vi "UHR-Fleezers Control (host) - 12.8.vi"() -> ()   [LabVIEW 2012] (continued)
        n3045 = xnode "Read/Write Control"("FPGA VI Reference In"=w4146, "error in"=w4145) -> ("FPGA VI Reference Out"=w4144:T20, "error out"=w4143:errorcluster, "APD 3 Gate Late Counter"=→"APD 3 Gate Late Counter":u8, "APD 3 Gate Relative Phase"=→"APD 3 Gate Relative Phase":i16)
      }
    }
    n3046 = Not Equal?(x=w3817, y="Calibration") -> (x != y?=w3778:bool)
    n3047 = case shown="True" w3778 {
      tunnel: w3815 -> [_ w4177]
      tunnel: w3814 -> [_ w4176]
      tunnel: w3813 -> [_ w4175]
      tunnel: w3810 -> [_ w4174]
      tunnel: w3754 -> [_ w4173]
      frame False {
      }
      frame True {
        n3048 = property on="Force" class="WFChart (strict)"("YScale.NameLbl.Text"=w4177) -> ()  [unwired: 2 in, 2 out]
        n3049 = property on="T2 X" class="DigNum (strict)"("Caption.Text"=w4175) -> ()  [unwired: 2 in, 2 out]
        n3050 = property on="T1 X" class="DigNum (strict)"("Caption.Text"=w4176) -> ()  [unwired: 2 in, 2 out]
        n3051 = property on="Mean" class="DigNum (strict)"("Caption.Text"=w4174) -> ()  [unwired: 2 in, 2 out]
        n3052 = property on="Difference" class="DigNum (strict)"("Caption.Text"=w4173) -> ()  [unwired: 2 in, 2 out]
      }
    }
    n3053 = Unbundle By Name(w3553) -> ("Y"=w3801:dbl[])
    n3054 = Unbundle By Name(w3552) -> ("Y"=w3804:dbl[])
    n3055 = Subtract(x=w3801, y=w3799) -> (x-y=w3802:dbl[])
    n3056 = Subtract(x=w3804, y=w3798) -> (x-y=w3803:dbl[])
    n3057 = Multiply(x=w3803, y="T2 alpha_x (nm/V)") -> (x*y=w3603:dbl[])
    n3058 = Multiply(x="T1 alpha_x (nm/V)", y=w3802) -> (x*y=w3604:dbl[])
    n3059 = Not(x="Trap Trig. Fl.") -> (.not. x?=w3640:bool)
    n3060 = Multiply(x=w3825, y=-1.0) -> (x*y=w3806:waveform(dbl))
    n3061 = Subtract(x=w3604, y=w3603) -> (x-y=w3796:dbl[])
    n3062 = Unbundle By Name(w3825) -> ("Y"=w3769:dbl[])
    n3063 = Unbundle By Name(w3826) -> ("Y"=w3605:dbl[])
    n3064 = Negate(x=w3796) -> (-x=w3601:dbl[])
    n3065 = Build Array(w3826, w3806) -> (→"Force":waveform(dbl)[])
    n3066 = Subtract(x=w3601, y="Offset (nm)") -> (x-y=w3768:dbl[])
    n3067 = call-poly <vilib>:"Mean.vi"("X"=w3769) -> ("mean"=w3607:dbl)  [unwired: 1 out]
    "T2 X" <- w3607
    n3068 = Negate(x=w3769) -> (-x=w3546:dbl[])
    n3069 = call-poly <vilib>:"Mean.vi"("X"=w3605) -> ("mean"=w3608:dbl)  [unwired: 1 out]
    "T1 X" <- w3608
    n3070 = Negate(x=w3607) -> (-x=w3606:dbl)
    n3071 = Bundle By Name(cluster=w3553, "Y"=w3768) -> (w3746:waveform(dbl))
    "Bead Separation" <- w3746
    n3072 = Add(x=w3605, y=w3546) -> (x+y=w3770:dbl[])
    n3073 = Divide(x=w3770, y=2.0) -> (x/y=w3549:dbl[])
    n3074 = Add(x=w3608, y=w3606) -> (x+y=w3812:dbl)
    n3075 = Subtract(x=w3608, y=w3606) -> (x-y=→"Difference":dbl)
    n3076 = Select(t=w3546, s="Only check fixed trap T2", f=w3549) -> (s? t:f=→"Vec Mean of T1 T2":dbl[])
    n3077 = Divide(x=w3812, y=2.0) -> (x/y=w3772:dbl)
    "Mean" <- w3772
    n3078 = feedback-in #25("Trap Trig. Fl.") -> ()
    n3079 = feedback #25("Trap Trig. Fl.") -> (w3638:bool)
    n3080 = And(x=w3640, y=w3638) -> (x .and. y?=w3639:bool)
    n3081 = case "If have just turned off triggering" shown="True" w3639 {
      tunnel: w3621 -> [_ w3974]
      tunnel: w3620 -> [_ w3973]
      frame False {
      }
      frame True {
        w3972 = FALSE ("FPGA Trap Trig")
        n3082 = xnode "Read/Write Control"("FPGA VI Reference In"=w3974, "error in"=w3973, "FPGA Trap Trig"=w3972) -> ("FPGA VI Reference Out"=w3971:T20, "error out"=w3970:errorcluster)
        n3083 = xnode "Read/Write Control"("FPGA VI Reference In"=w3971, "error in"=w3970, "TTrig?"=w3972) -> ()  [unwired: 2 out]
        n3084 = local write "Initializing"(FALSE ("Initializing")) -> ()
        n3085 = local write "Triggered"(FALSE ("Triggered")) -> ()
        n3086 = local write "Waiting"(FALSE ("Waiting")) -> ()
      }
    }
    n3087 = Not(x=w3638) -> (.not. x?=w3651:bool)
    n3088 = And(x="Trap Trig. Fl.", y=w3651) -> (x .and. y?=w3648:bool)
    n3089 = local read "Tether"() -> (w3773:bool)
    n3090 = Or(x=w3648, y="Reinitialize") -> (x .or. y?=w3634:bool)
    n3091 = feedback #26(w3644) -> (w3649:string)
    n3092 = Select(t=w3644, s=w3648, f=w3649) -> (s? t:f=w3643:string)
    n3093 = Select(t=w3644, s="Reinitialize", f=w3643) -> (s? t:f=w3642:string)
    n3094 = feedback #27(0) -> (w3646:i32)
    n3095 = feedback #28(w3768) -> (w3767:dbl[])
    n3096 = Build Array (concatenate)(w3768, w3767) -> (w3602:dbl[])
    n3097 = case "For determining if there is a tether still" shown="True" w3773 {
      tunnel: w3772 -> [_ w4098]
      frame False {
      }
      frame True {
        n3098 = Greater?(x="Lost Tether Alarm Threshold (pN)", y=w4098) -> (0:w4096:bool)
        n3099 = case shown="True" w4096 {
          frame False {
          }
          frame True {
            w4099 = FALSE ("Value (Signaling)")
            n3100 = flat-sequence {
              frame #0 {
                # "stop only if saving"
                n3101 = local read "Saving..."() -> (w4111:bool)
                n3102 = And(x=w4111, y="TA Cancel Save?") -> (x .and. y?=w4110:bool)
                n3103 = local write "Stop Saving"(w4110) -> ()
              }
              frame #1 {
                n3104 = case shown="True" "TA Green Off?" {
                  frame False {
                  }
                  frame True {
                    w4114 = FALSE ("Fl. Triggered...")
                    n3105 = local write "Fl. Triggered..."(w4114) -> ()
                    n3106 = property on="Green Laser ON" class="Bool (strict)"("Val(Sgnl)"=w4114) -> ()  [unwired: 2 in, 2 out]
                  }
                }
              }
            }
            n3107 = local read "Time tether formed"() -> (w4105:timestamp)
            n3108 = Get Date/Time In Seconds() -> (seconds since 1Jan1904=w4106:timestamp)
            n3109 = Subtract(x=w4106, y=w4105) -> (x-y=w4104:dbl)
            n3110 = Number To Decimal String(number=w4104) -> (decimal integer string=w4101:string)  [unwired: 1 out]
            n3111 = local read "Messages"() -> (w4108:string)
            n3112 = call <vilib>:"Beep.vi"() -> ()  [unwired: 3 in, 9 out]
            n3113 = Concatenate Strings("Lost tether (" ("Message to add"), w4101, " s)." ("string")) -> (w4103:string)
            n3114 = local write "Tether"(FALSE ("Tether")) -> ()
            n3115 = call "Update messages.vi"("Message to add"=w4103, "Old message string"=w4108) -> ("New message string"=w4107:string)
            n3116 = local write "Messages"(w4107) -> ()
            n3117 = property on="Fl. Triggered..." class="Bool (strict)"("Val(Sgnl)"=w4099) -> ()  [unwired: 2 in, 2 out]
            n3118 = local write "Dip for Protein"(w4099) -> ()
            n3119 = property on="Trap Pos. FB ON" class="Bool (strict)"("Val(Sgnl)"=w4099) -> ()  [unwired: 2 in, 2 out]
            n3120 = property on="Trap Trig. Fl." class="Bool (strict)"("Val(Sgnl)"=w4099) -> ()  [unwired: 2 in, 2 out]
          }
        }
      }
    }
    n3121 = case "For triggering actions based on the trap position (e.g., turning the excitation laser on if trap under feedback moves so far)" shown="True" "Trap Trig. Fl." {
      tunnel: w3629 -> [_ w3987]
      tunnel: w3642 -> [_ w3986]
      tunnel: ["" ("t") w3985] -> w3650
      tunnel: w3634 -> [_ w3984]
      tunnel: [0 ("t") w3983] -> w3647
      tunnel: w3646 -> [_ w3982]
      tunnel: w3621 -> [_ w3981]
      tunnel: w3620 -> [_ w3980]
      frame False {
      }
      frame True {
        n3122 = case shown="\"Wait for trigger\"" w3986 {
          tunnel: w3987 -> [w4004 _ _ w4052]
          tunnel: [w4001 w4033 "" ("t") w4055] -> w3985
          tunnel: w3984 -> [_ _ _ w4043]
          tunnel: [w4000 w4030 0 ("t") w4044] -> w3983
          tunnel: w3982 -> [_ w4032 _ w4050]
          tunnel: w3981 -> [w3989 w4027 _ w4046]
          tunnel: w3980 -> [w3988 w4026 _ w4045]
          frame "Wait for trigger" {
            n3123 = local read "Trap Trig. (FPGA)"() -> (w3992:bool)
            n3124 = Subtract(x=w4004, y="Mean T1 Position\nto compare (nm)") -> (x-y=w3997:dbl[])
            n3125 = call <vilib>:"Std Deviation and Variance.vi"("X"=w3997) -> ("mean"=→"mean":dbl, "standard deviation"=→"standard\ndeviation":dbl)  [unwired: 1 in, 1 out]
            n3126 = Array Max & Min(array=w3997) -> (max value=→"max value":dbl, min value=→"min value":dbl)  [unwired: 2 out]
            n3127 = Greater?(x=w3997, y="Threshold (nm)") -> (0:w4007:bool[])
            n3128 = case shown="True" w3992 {
              tunnel: w3989 -> [_ w4013]
              tunnel: w3988 -> [_ w4012]
              tunnel: [FALSE ("TTrig?") w4011] -> w3995
              frame False {
              }
              frame True {
                n3129 = xnode "Read/Write Control"("FPGA VI Reference In"=w4013, "error in"=w4012) -> ("TTrig?"=w4011:bool)  [unwired: 2 out]
              }
            }
            n3130 = Or Array Elements(Boolean array=w4007) -> (logical OR=w3994:bool)
            n3131 = Select(t=w3995, s=w3992, f=w3994) -> (s? t:f=w3993:bool)
            n3132 = Not(x=w3992) -> (.not. x?=w3991:bool)
            n3133 = And(x=w3993, y=w3991) -> (x .and. y?=w3990:bool)
            n3134 = Select(t="Triggered", s=w3993, f="Wait for trigger") -> (s? t:f=w4001:string)
            n3135 = case shown="True" w3993 {
              tunnel: [0 0] -> w4000
              tunnel: w3989 -> [_ w4018]
              tunnel: w3988 -> [_ w4017]
              frame False {
                "Waiting" <- TRUE ("Waiting")
              }
              frame True {
                n3136 = xnode "Read/Write Control"("FPGA VI Reference In"=w4018, "error in"=w4017, "TTrig?"=FALSE) -> ()  [unwired: 2 out]
                n3137 = local read "Messages"() -> (w4021:string)
                n3138 = call <vilib>:"Beep.vi"() -> ()  [unwired: 12 in]
                n3139 = call "Update messages.vi"("Message to add"="Unwinding trigger.", "Old message string"=w4021) -> ("New message string"=w4022:string)
                n3140 = local write "Messages"(w4022) -> ()
                n3141 = local write "Waiting"(FALSE ("Waiting")) -> ()
                "Triggered" <- TRUE ("Triggered")
              }
            }
            n3142 = case "Only need to turn on laser if host triggered" shown="True" w3990 {
              frame False {
              }
              frame True {
                n3143 = property on="Green Laser ON" class="Bool (strict)"("Val(Sgnl)"=TRUE ("Value (Signaling)")) -> ()  [unwired: 2 in, 2 out]
              }
            }
          }
          frame "Triggered" {
            n3144 = local read "Trap Trig. (FPGA)"() -> (w4029:bool)
            n3145 = Increment(x=w4032) -> (x+1=w4030:i32)
            n3146 = Greater Or Equal?(x=w4030, y="Fl. ON time (n)") -> (x >= y?=w4028:bool)
            n3147 = Select(t="Wait for trigger", s=w4028, f="Triggered" ("t")) -> (s? t:f=w4033:string)
            n3148 = And(x=w4028, y=w4029) -> (x .and. y?=w4025:bool)
            n3149 = case shown="True" w4025 {
              tunnel: w4027 -> [_ w4037]
              tunnel: w4026 -> [_ w4036]
              frame False {
              }
              frame True {
                n3150 = xnode "Read/Write Control"("FPGA VI Reference In"=w4037, "error in"=w4036, "FPGA Trap Trig"=TRUE) -> ()  [unwired: 2 out]
              }
            }
            n3151 = case shown="True" w4028 {
              frame False {
              }
              frame True {
                w4039 = FALSE ("Value (Signaling)")
                n3152 = local write "Triggered"(w4039) -> ()
                n3153 = local write "Waiting"(TRUE ("Waiting")) -> ()
                n3154 = property on="Green Laser ON" class="Bool (strict)"("Val(Sgnl)"=w4039) -> ()  [unwired: 2 in, 2 out]
              }
            }
          }
          frame "Do nothing" {
          }
          frame "Initialize", Default {
            n3155 = Increment(x=w4050) -> (x+1=w4054:i32)
            n3156 = Select(t=1, s=w4043, f=w4054) -> (s? t:f=w4044:i32)
            n3157 = feedback #29(w4052) -> (w4058:dbl[])
            n3158 = Build Array (concatenate)(w4052, w4058) -> (w4051:dbl[])
            n3159 = Greater Or Equal?(x=w4044, y="Wait to get offset (n)") -> (x >= y?=w4047:bool)
            n3160 = Select(t=w4052, s=w4043, f=w4051) -> (s? t:f=w4053:dbl[])
            n3161 = feedback-in #29(w4053) -> ()
            n3162 = call-poly <vilib>:"Mean.vi"("X"=w4053) -> ("mean"=w4048:dbl)  [unwired: 1 out]
            n3163 = local write "Mean T1 Position\nto compare (nm)"(w4048) -> ()
            n3164 = case shown="True" w4043 {
              tunnel: w4046 -> [_ w4064]
              tunnel: w4045 -> [_ w4063]
              frame False {
              }
              frame True {
                w4060 = FALSE ("FPGA Trap Trig")
                n3165 = xnode "Read/Write Control"("FPGA VI Reference In"=w4064, "error in"=w4063, "FPGA Trap Trig"=w4060) -> ("FPGA VI Reference Out"=w4062:T20, "error out"=w4061:errorcluster)
                n3166 = xnode "Read/Write Control"("FPGA VI Reference In"=w4062, "error in"=w4061, "TTrig?"=w4060) -> ()  [unwired: 2 out]
              }
            }
            n3167 = Select(t="Wait for trigger", s=w4047, f="Initialize") -> (s? t:f=w4055:string)
            n3168 = case shown="True" w4047 {
              tunnel: w4048 -> [_ w4067]
              tunnel: w4046 -> [_ w4076]
              tunnel: w4045 -> [_ w4075]
              frame False {
                n3169 = local write "Waiting"(FALSE ("Waiting")) -> ()
                "Initializing" <- TRUE ("Initializing")
              }
              frame True {
                n3170 = local read "Threshold (nm)"() -> (w4079:dbl)
                n3171 = local read "AOM X Cal (nm/MHz)"() -> (w4078:dbl)
                n3172 = Add(x=w4067, y=w4079) -> (x+y=w4080:dbl)
                n3173 = Divide(x=w4080, y=w4078) -> (x/y=w4077:dbl)
                n3174 = call "IR AOM freq to word.vi"("Frequency In (MHz)"=w4077) -> ("Frequency Word Out (double)"=w4074:dbl)
                n3175 = local write "Initializing"(FALSE ("Initializing")) -> ()
                n3176 = local write "Waiting"(TRUE ("Waiting")) -> ()
                n3177 = To Quad Integer(1:w4074) -> (0:w4073:i64)
                n3178 = xnode "Read/Write Control"("FPGA VI Reference In"=w4076, "error in"=w4075, "FPGA TTrig Thresh"=w4073) -> ("FPGA VI Reference Out"=w4070:T20, "error out"=w4069:errorcluster)
                n3179 = xnode "Read/Write Control"("FPGA VI Reference In"=w4070, "error in"=w4069, "FPGA Trap Trig"=TRUE) -> ()  [unwired: 2 out]
              }
            }
          }
        }
      }
    }
    n3180 = feedback-in #26(w3650) -> ()
    n3181 = feedback-in #27(w3647) -> ()
    n3182 = Split 1D Array(array=w3602, index=w3664) -> (first subarray=w3764:dbl[])  [unwired: 1 out]
    n3183 = feedback-in #28(w3764) -> ()
    n3184 = call-poly <vilib>:"Mean.vi"("X"=w3764) -> ("mean"=w3763:dbl)  [unwired: 1 out]
    "Bead Mean (nm)" <- w3763
    n3185 = Subtract(x=w3764, y=w3763) -> (x-y=w3762:dbl[])
    n3186 = Square(x=w3762) -> (x^2=w3761:dbl[])
    n3187 = call-poly <vilib>:"Mean.vi"("X"=w3761) -> ("mean"=w3760:dbl)  [unwired: 1 out]
    n3188 = Square Root(x=w3760) -> (sqrt(x)=w3759:dbl)
    n3189 = Multiply(x=10.0, y=w3759) -> (x*y=→"RMS (Ang)":dbl)
    n3190 = xnode ("Read/Write Control")("FPGA VI Reference In"=w3794, "error in"=w3793) -> ("FPGA VI Reference Out"=w3632:T20, "error out"=w3631:errorcluster, "AI2 Y Sum Set 1"=w3887:i16, "AI2 Y Sum Set 2"=w3886:i16, "AI1 X Set 1"=w3696:fxp<+/-,16,1>, "AI1 X Set 2"=w3695:fxp<+/-,16,1>, "Trap Pos FB Int Signal"=→"Trap Pos FB Int Signal":fxp<+/-,24,9>, "Trap Pos FB Int-Norm Signal"=→"Trap Pos FB Int-Norm Signal":fxp<+/-,16,1>, "Trap Pos FB Action"=w3689:i64, "Scanning"=→"AOD Scanning":bool, "Scan I"=→"AOD Scan I":u64, "Scanning MCL"=w3889:bool, "Scan I (MCL)"=→"MCL Scan I":u64, "Green FB Sum"=w3829:i16, "Trap Pos FB Action"=w3619:i64, "TTrig Fin Thresh"=w3615:i64, "Red FB Intensity"=w3596:i16, "Blue Intensity"=w3591:i16)
    "MCL Scanning" <- w3889
    "Trap Pos FB Action" <- w3689
    n3191 = Divide(x=w3596, y=3276.7) -> (x/y=w3595:dbl)
    "Red laser intensity (V)" <- w3595
    n3192 = Divide(x=w3591, y=3276.7) -> (x/y=w3590:dbl)
    "Blue laser intensity (V)" <- w3590
    n3193 = Divide(x=w3829, y=3276.7) -> (x/y=w3594:dbl)
    "Green laser intensity (V)" <- w3594
    n3194 = local read "FB Trig Integrate"() -> (w3613:u32)
    n3195 = Divide(x=w3619, y=w3613) -> (x/y=w3612:dbl)
    "TTrig Sig (Int)" <- w3612
    n3196 = Bundle(w3594, w3595, w3590) -> (→"Fluorescence laser intensities plot":cluster{dbl, dbl, dbl})  [unwired: 1 in]
    n3197 = Divide(x=w3615, y=w3613) -> (x/y=w3610:dbl)
    "TTrig Fin Thresh (Int)" <- w3610
    n3198 = local read "AOM X Cal (nm/MHz)"() -> (w3618:dbl)
    n3199 = local read "AI2 (V)"() -> (w3888:cluster{"Set 1":dbl, "Set 2":dbl})
    n3200 = Bundle By Name(cluster=w3888, "Set 1"=w3887, "Set 2"=w3886) -> (w3884:cluster{"Set 1":dbl, "Set 2":dbl})
    n3201 = Divide(x=w3689, y=327.67) -> (x/y=→"Action (%)":dbl)
    n3202 = local read "Trap X (AI1)"() -> (w3709:T10)
    n3203 = call "IR AOM word double to freq.vi"("Frequency Word In (double)"=w3610) -> ("Frequency Out (MHz)"=w3609:dbl)
    n3204 = call "IR AOM word double to freq.vi"("Frequency Word In (double)"=w3612) -> ("Frequency Out (MHz)"=w3611:dbl)
    n3205 = Divide(x=w3884, y=3276.7) -> (x/y=w3883:cluster{"Set 1":dbl, "Set 2":dbl})
    n3206 = Multiply(x=w3611, y=w3618) -> (x*y=w3617:dbl)
    "TTrig Sig (nm)" <- w3617
    n3207 = Multiply(x=w3609, y=w3618) -> (x*y=w3616:dbl)
    "TTrig Fin Thresh (nm)" <- w3616
    n3208 = local write "AI2 (V)"(w3883) -> ()
    n3209 = Bundle(cluster=w3709, "Trap 1"=w3696, "Trap 2"=w3695) -> (→"Trap X (AI1)":T10)
    n3210 = Bundle(w3617, w3616) -> (→"TTrig":cluster{dbl, dbl})  [unwired: 1 in]
    n3211 = flat-sequence "To save data" {
      tunnel: [w4998] -> w3907
      tunnel: [w4999] -> w3906
      tunnel: w3858 -> [w4992]
      tunnel: w3637 -> [w4996]
      tunnel: ["Save Calibration"] -> w3880
      tunnel: w3877 -> [w4995]
      tunnel: [w4988] -> w3876
      tunnel: [w4985] -> w3875
      tunnel: [w4982] -> w3874
      tunnel: w3857 -> [w4984]
      tunnel: w3776 -> [w4978]
      tunnel: [w4978] -> w3775
      tunnel: [w4970] -> w3747
      tunnel: [w4973] -> w3677
      tunnel: [w4972] -> w3676
      tunnel: w3907 -> [w5248]
      tunnel: w3906 -> [w5247]
      tunnel: w3678 -> [w5246]
      tunnel: w3880 -> [w5245]
      tunnel: w3876 -> [w5243]
      tunnel: w3875 -> [w5242]
      tunnel: w3874 -> [w5241]
      tunnel: w3756 -> [w5240]
      tunnel: w3786 -> [w5239]
      tunnel: w3775 -> [w5238]
      tunnel: w3747 -> [w5237]
      tunnel: w3746 -> [w5236]
      tunnel: w3576 -> [w5235]
      tunnel: w3677 -> [w5234]
      tunnel: w3676 -> [w5233]
      tunnel: w3675 -> [w5232]
      tunnel: w3598 -> [w5231]
      frame #0 {
        n3212 = Or(x="Start Saving", y="Start saving data + video") -> (x .or. y?=w4970:bool)
        n3213 = case shown="True" "Start saving data + video" {
          frame False {
          }
          frame True {
            n3214 = stacked-sequence {
              frame #0 {
                n3215 = local write "New Video File"(TRUE ("New Video File")) -> ()
              }
              frame #1 {
                n3216 = local write "Save Video"(TRUE ("Save Video")) -> ()
              }
            }
          }
        }
        n3217 = Or(x="Save N Sets", y=w4970) -> (x .or. y?=w4979:bool)
        n3218 = To Double Precision Float(number=w4995) -> (double precision float=w4989:dbl)
        n3219 = Build Array(w4979, "Save Calibration", w4992, w4984) -> (w4994:bool[])
        n3220 = Compound Arithmetic op=OR("Save Calibration", w4992, w4979, w4984) -> (w4997:bool)
        n3221 = Boolean Array To Number(Boolean array=w4994) -> (number=w4991:u32)
        n3222 = feedback #30(FALSE ("Save APD Data\nwith Trap Data")) -> (w4974:bool)
        n3223 = feedback #31(refnum<k0> refnum) -> (w5000:refnum<file>)
        n3224 = feedback #32(refnum<k0> refnum) -> (w4976:refnum<file>)
        n3225 = feedback #33(FALSE ("Save APD Data\nwith Trap Data")) -> (w4983:bool)
        n3226 = feedback #34(refnum<k0> refnum) -> (w4986:refnum<file>)
        n3227 = feedback #35(0) -> (w5002:i32)
        n3228 = feedback #36() -> (w4990:u32)  [unwired: 1 out]
        n3229 = case shown="True" w4997 {
          tunnel: [w5011 1] -> w4998
          tunnel: w5002 -> [w5013 _]
          tunnel: [w5012 w5044] -> w4999
          tunnel: w5000 -> [w5012 _]
          tunnel: w4996 -> [_ w5062]
          tunnel: w4989 -> [_ w5060]
          tunnel: w4991 -> [_ w5063]
          tunnel: [w5010 w5043] -> w4988
          tunnel: w4990 -> [w5010 _]
          tunnel: [w5009 w5041] -> w4985
          tunnel: w4986 -> [w5009 _]
          tunnel: [w5008 w5040] -> w4982
          tunnel: w4983 -> [w5008 _]
          tunnel: w4970 -> [_ w5038]
          tunnel: w4978 -> [_ w5037]
          tunnel: [w5007 w5029] -> w4972
          tunnel: w4976 -> [w5007 _]
          tunnel: [w5006 w5028] -> w4973
          tunnel: w4974 -> [w5006 _]
          frame False {
            n3230 = Increment(x=w5013) -> (x+1=w5011:i32)
          }
          frame True {
            w5034 = FALSE ("Start Saving")
            w5039 = 9.0  # File Version
            w5046 = FALSE ("prepend array or string size? (T)")
            w5045 = T28."big-endian, network order" ("byte order (0:big-endian, network order)")
            n3231 = local read "BD 1 Frequency 1 (MHz)"() -> (w5059:dbl)
            n3232 = local read "BD 2 Frequency 1 (MHz)"() -> (w5058:dbl)
            n3233 = local read "BD 1 Frequency 2 (MHz)"() -> (w5057:dbl)
            n3234 = local read "BD 2 Frequency 2 (MHz)"() -> (w5056:dbl)
            n3235 = local read "BD 1 Frequency 3 (MHz)"() -> (w5055:dbl)
            n3236 = local read "BD 2 Frequency 3 (MHz)"() -> (w5054:dbl)
            n3237 = Array Size(array=w5037) -> (size(s)=w5036:i32)
            n3238 = To Double Precision Float(number=w5036) -> (double precision float=w5035:dbl)
            n3239 = local write "Save Calibration"(w5034) -> ()
            n3240 = local write "Start Saving"(w5034) -> ()
            n3241 = Build Array("Save APD Data\nwith Trap Data", "Save Trap Pos. Data") -> (w5031:bool[])
            n3242 = Boolean Array To Number(Boolean array=w5031) -> (number=w5030:u32)
            n3243 = Build Array(w5059, w5058, w5057, w5056, w5055, w5054) -> (w5053:dbl[])
            n3244 = case shown="1, Default" w5063 {
              tunnel: w5062 -> [w5135 w5155 w5171 w5209]
              tunnel: w5035 -> [w5140 w5162 w5191 w5228]
              tunnel: w5060 -> [w5139 w5161 w5190 w5227]
              tunnel: [w5136 w5157 w5182 w5219] -> w5051
              tunnel: [w5127 "Cal sets to save" w5172 w5210] -> w5043
              tunnel: w5053 -> [w5137 w5158 w5184 w5221]
              tunnel: "Save APD Data\nwith Trap Data" -> [w5134 _ w5168 w5207]
              tunnel: [w5134 w5149 w5168 w5207] -> w5040
              tunnel: w5039 -> [w5130 w5150 w5166 w5205]
              tunnel: w5038 -> [w5129 _ _ _]
              tunnel: [w5120 w5149 w5165 w5195] -> w5028
              tunnel: "Save Trap Pos. Data" -> [w5120 _ w5165 w5195]
              tunnel: w5030 -> [w5119 _ w5164 w5194]
              frame 1, Default {
                # "timeseries"
                n3245 = case shown="True" "Profile" {
                  tunnel: [w5143 w5147] -> w5124
                  tunnel: [w5143 w5146] -> w5123
                  tunnel: [w5143 w5145] -> w5122
                  tunnel: [w5143 w5144] -> w5121
                  frame False {
                    w5143 = 0.0 ("f")
                  }
                  frame True {
                    n3246 = local read "Current Position"() -> (w5148:cluster{dbl, dbl, dbl})
                    n3247 = local read "Y change (mm)"() -> (w5144:dbl)
                    n3248 = Unbundle(w5148) -> (w5147:dbl, w5146:dbl, w5145:dbl)
                  }
                }
                n3249 = local read "Save ave N"() -> (w5142:dbl)
                n3250 = Multiply(x=w5142, y=w5135) -> (x*y=w5141:dbl)
                n3251 = To Double Precision Float(number=w5119) -> (double precision float=w5133:dbl)
                n3252 = Build Array(w5130, w5135, w5141, w5140, w5139, 0.0 ("f")) -> (w5138:dbl[])
                n3253 = Build Array(w5133, w5124, w5123, w5122, w5121) -> (w5131:dbl[])
                n3254 = Select(t=u32 4000000000, s=w5129, f="N sets to save") -> (s? t:f=w5127:u32)
                n3255 = Build Array (concatenate)(w5138, w5137, w5131) -> (w5136:dbl[])
              }
              frame 2 {
                w5152 = 0.0 ("f")
                w5149 = FALSE ("Save APD Data\nwith Trap Data")
                # "calibration"
                n3256 = Boolean To (0,1)(Boolean=w5149) -> (0, 1=w5154:i16)
                n3257 = To Double Precision Float(number=w5154) -> (double precision float=w5153:dbl)
                n3258 = Build Array(w5153, w5152, w5152, w5152, w5152) -> (w5151:dbl[])
                n3259 = Build Array(w5150, w5155, w5155, w5162, w5161, 1.0 ("t")) -> (w5159:dbl[])
                n3260 = Build Array (concatenate)(w5159, w5158, w5151) -> (w5157:dbl[])
                "Calibrating Trap..." <- TRUE ("Calibrating...")
              }
              frame 4 {
                w5169 = 0.0 ("f")
                # "scan dir (x/y = 0/1)"
                # "cycles/step"
                # "n scans (f/b)"
                # "steps"
                # "freq. range"
                # "AOD raster scan"
                n3261 = local read "Number of F/B Scans (AOD)"() -> (w5176:u16)
                n3262 = local read "Cycles/step (AOD)"() -> (w5178:u64)
                n3263 = local read "Scan Range (MHz)"() -> (w5181:dbl)
                n3264 = local read "Scan steps (AOD)"() -> (w5180:u64)
                n3265 = local read "Scan BD"() -> (w5188:bool)
                n3266 = local read "Save ave N"() -> (w5193:dbl)
                n3267 = Boolean To (0,1)(Boolean=w5188) -> (0, 1=w5187:i16)
                n3268 = To Double Precision Float(number=w5176) -> (double precision float=w5175:dbl)
                n3269 = To Double Precision Float(number=w5180) -> (double precision float=w5179:dbl)
                n3270 = To Double Precision Float(number=w5178) -> (double precision float=w5177:dbl)
                n3271 = To Double Precision Float(number=w5187) -> (double precision float=w5186:dbl)
                n3272 = Multiply(x=w5193, y=w5171) -> (x*y=w5192:dbl)
                n3273 = To Double Precision Float(number=w5164) -> (double precision float=w5170:dbl)
                n3274 = Build Array(w5170, w5169, w5169, w5169, w5169) -> (w5167:dbl[])
                n3275 = local read "N sets should be saved"() -> (w5173:dbl)
                n3276 = Build Array(w5186, w5181, w5179, w5177, w5175) -> (w5183:dbl[])
                n3277 = Build Array(w5166, w5171, w5192, w5191, w5190, 2.0 ("t")) -> (w5185:dbl[])
                n3278 = Round Toward +Infinity(x=w5173) -> (ceil(x): smallest int >= x=w5174:dbl)
                n3279 = Build Array (concatenate)(w5185, w5184, w5167, w5183) -> (w5182:dbl[])
                n3280 = To Unsigned Long Integer(number=w5174) -> (unsigned 32bit integer=w5172:u32)
              }
              frame 8 {
                w5202 = 0.0 ("f")
                # "MCL raster scan"
                n3281 = local read "Number of scans (MCL)"() -> (w5197:u64)
                n3282 = local read "Scan lines (y)"() -> (w5196:u64)
                n3283 = local read "2D or 1D Scan"() -> (w5199:bool)
                n3284 = local read "Scan Range (V)\n(of steps)"() -> (w5218:dbl)
                n3285 = local read "Fast Scan Dir"() -> (w5225:bool)
                n3286 = local read "Cycles/step (MCL)"() -> (w5215:u64)
                n3287 = local read "Scan steps (MCL)"() -> (w5217:u64)
                n3288 = Select(t=w5196, s=w5199, f=w5197) -> (s? t:f=w5198:u64)
                n3289 = Boolean To (0,1)(Boolean=w5199) -> (0, 1=w5201:i16)
                n3290 = local read "Save ave N"() -> (w5230:dbl)
                n3291 = local read "Initial X"() -> (w5204:dbl)
                n3292 = local read "Initial Y"() -> (w5203:dbl)
                n3293 = To Double Precision Float(number=w5201) -> (double precision float=w5200:dbl)
                n3294 = Boolean To (0,1)(Boolean=w5225) -> (0, 1=w5224:i16)
                n3295 = To Double Precision Float(number=w5198) -> (double precision float=w5213:dbl)
                n3296 = To Double Precision Float(number=w5217) -> (double precision float=w5216:dbl)
                n3297 = To Double Precision Float(number=w5215) -> (double precision float=w5214:dbl)
                n3298 = To Double Precision Float(number=w5224) -> (double precision float=w5223:dbl)
                n3299 = Multiply(x=w5230, y=w5209) -> (x*y=w5229:dbl)
                n3300 = To Double Precision Float(number=w5194) -> (double precision float=w5208:dbl)
                n3301 = local read "N sets should be saved (MCL)"() -> (w5211:dbl)
                n3302 = Build Array(w5208, w5200, w5202, w5202, w5202) -> (w5206:dbl[])
                n3303 = Build Array(w5223, w5218, w5216, w5214, w5213, w5204, w5203) -> (w5220:dbl[])
                n3304 = Build Array(w5205, w5209, w5229, w5228, w5227, 3.0 ("t")) -> (w5222:dbl[])
                n3305 = Round Toward +Infinity(x=w5211) -> (ceil(x): smallest int >= x=w5212:dbl)
                n3306 = Build Array (concatenate)(w5222, w5221, w5206, w5220) -> (w5219:dbl[])
                n3307 = To Unsigned Long Integer(number=w5212) -> (unsigned 32bit integer=w5210:u32)
              }
            }
            n3308 = local read "Index"() -> (w5068:dbl)
            n3309 = call "Create new save file.vi"("Insert"="", "Ext"=".dat", "Index In"=w5068) -> ("Path Out"=w5024:path, "Index Out"=w5042:dbl)
            n3310 = local write "Save file name"(w5024) -> ()
            n3311 = local write "Index"(w5042) -> ()
            n3312 = local write "Save index"(w5042) -> ()
            n3313 = Array Size(array=w5051) -> (size(s)=w5052:i32)
            n3314 = Open/Create/Replace File(file path (use dialog)=w5024, operation (0:open)=T29."create", access (0:read/write)=enum16{"read/write", "read-only", "write-only"}."write-only") -> (refnum out=w5065:refnum<file>)  [unwired: 1 in, 4 out]
            n3315 = local write "Saving..."(TRUE ("Saving...")) -> ()
            n3316 = To Double Precision Float(number=w5052) -> (double precision float=w5050:dbl)
            n3317 = String Length(string="Comment (data description)") -> (length=w5049:i32)
            n3318 = To Double Precision Float(number=w5049) -> (double precision float=w5048:dbl)
            n3319 = Deny Access(7:w5065) -> (3:w5064:refnum<file>)  [unwired: 1 in, 2 out]
            n3320 = Build Array (concatenate)(w5050, w5051, w5048) -> (w5023:dbl[])
            n3321 = case "If fluorescence data to be saved" shown="True" w5040 {
              tunnel: w5024 -> [_ w5118]
              tunnel: [refnum<k0> refnum w5098] -> w5041
              frame False {
              }
              frame True {
                w5097 = 0.0
                n3322 = local read "APD Integration Time (s)"() -> (w5103:dbl)
                n3323 = local read "N APD Samp/step"() -> (w5096:dbl)
                n3324 = local read "Number of APDs"() -> (w5095:u8)
                n3325 = Path To String(path=w5118) -> (string=w5117:string)
                n3326 = String Length(string=w5117) -> (length=w5116:i32)
                n3327 = Subtract(x=w5116, y=4) -> (x-y=w5114:i32)
                n3328 = String Subset(string=w5117, length (rest)=w5114) -> (substring=w5113:string)  [unwired: 1 out]
                n3329 = Build Array(w5103, w5096, w5095, w5097, w5097, w5097, w5097, w5097) -> (w5100:dbl[])
                n3330 = Concatenate Strings(w5113, "_fl.dat" ("string")) -> (w5111:string)
                n3331 = Array Size(array=w5100) -> (size(s)=w5102:i32)
                n3332 = String To Path(string=w5111) -> (path=w5107:path)
                n3333 = Open/Create/Replace File(file path (use dialog)=w5107, operation (0:open)=T29."create", access (0:read/write)=enum16{"read/write", "read-only", "write-only"}."write-only") -> (refnum out=w5108:refnum<file>)  [unwired: 1 in, 4 out]
                n3334 = Deny Access(7:w5108) -> (3:w5104:refnum<file>)  [unwired: 1 in, 2 out]
                n3335 = To Double Precision Float(number=w5102) -> (double precision float=w5101:dbl)
                n3336 = Build Array (concatenate)(w5101, w5100) -> (w5099:dbl[])
                n3337 = Write to Binary File(file (use dialog)=w5104, data=w5099, 5:FALSE ("prepend array or string size? (T)"), 9:T28."big-endian, network order" ("byte order (0:big-endian, network order)")) -> (refnum out=w5098:refnum<file>)  [unwired: 1 in, 3 out]
              }
            }
            n3338 = case shown="True" w5028 {
              tunnel: w5024 -> [_ w5079]
              tunnel: [refnum<k0> refnum w5078] -> w5029
              frame False {
              }
              frame True {
                w5074 = 0.0 ("element")
                n3339 = Path To String(path=w5079) -> (string=w5093:string)
                n3340 = Build Array(w5074, w5074, w5074, w5074, w5074, w5074, w5074, w5074) -> (w5075:dbl[])
                n3341 = String Length(string=w5093) -> (length=w5092:i32)
                n3342 = Subtract(x=w5092, y=4) -> (x-y=w5090:i32)
                n3343 = Array Size(array=w5075) -> (size(s)=w5077:i32)
                n3344 = String Subset(string=w5093, length (rest)=w5090) -> (substring=w5089:string)  [unwired: 1 out]
                n3345 = To Double Precision Float(number=w5077) -> (double precision float=w5076:dbl)
                n3346 = Concatenate Strings(w5089, "_pos.dat" ("string")) -> (w5087:string)
                n3347 = Build Array (concatenate)(w5076, w5075) -> (w5073:dbl[])
                n3348 = String To Path(string=w5087) -> (path=w5083:path)
                n3349 = Open/Create/Replace File(file path (use dialog)=w5083, operation (0:open)=T29."create", access (0:read/write)=enum16{"read/write", "read-only", "write-only"}."write-only") -> (refnum out=w5084:refnum<file>)  [unwired: 1 in, 4 out]
                n3350 = Deny Access(7:w5084) -> (3:w5080:refnum<file>)  [unwired: 1 in, 2 out]
                n3351 = Write to Binary File(file (use dialog)=w5080, data=w5073, 5:FALSE ("prepend array or string size? (T)"), 9:T28."big-endian, network order" ("byte order (0:big-endian, network order)")) -> (refnum out=w5078:refnum<file>)  [unwired: 1 in, 3 out]
              }
            }
            n3352 = Write to Binary File(file (use dialog)=w5064, data=w5023, 5:w5046, 9:w5045) -> (refnum out=w5047:refnum<file>)  [unwired: 1 in, 3 out]
            n3353 = Write to Binary File(file (use dialog)=w5047, data="Comment (data description)", 5:w5046, 9:w5045) -> (refnum out=w5044:refnum<file>)  [unwired: 1 in, 3 out]
            n3354 = local read "connection reference"() -> (w5026:T17)
            n3355 = Bundle("Comment (data description)"="Comment (data description)", "Channel 1 Buffer"="Channel 1 Buffer", "Channel 2 Buffer"="Channel 2 Buffer", "Channel 3 Buffer"="Channel 3 Buffer", "Title"="Title", "DNA Construct"="DNA Construct", "Bead diameter"="Bead diameter", "Name"="Name") -> (w5014:T50)  [unwired: 1 in]
            n3356 = call "MattFileCreator-v9.vi"("Comments"=w5014, "Input Array"=w5023, "File path"=w5024, "table"="labview", "connection reference"=w5026) -> ("connection reference out"=w5025:T17)  [unwired: 5 in, 1 out]
            n3357 = local write "connection reference"(w5025) -> ()
          }
        }
        n3358 = feedback-in #30(w4973) -> ()
        n3359 = feedback-in #31(w4999) -> ()
        n3360 = feedback-in #32(w4972) -> ()
        n3361 = feedback-in #33(w4982) -> ()
        n3362 = feedback-in #34(w4985) -> ()
        n3363 = feedback-in #35(w4998) -> ()
        n3364 = feedback-in #36(w4988) -> ()
      }
      frame #1 {
        n3365 = local read "Saving..."() -> (w5244:bool)
        n3366 = case shown="True" w5244 {
          tunnel: w5248 -> [_ w5260]
          tunnel: w5247 -> [_ w5274]
          tunnel: w5246 -> [_ w5270]
          tunnel: w5245 -> [_ w5269]
          tunnel: w5243 -> [_ w5268]
          tunnel: w5242 -> [_ w5263]
          tunnel: w5241 -> [_ w5262]
          tunnel: w5240 -> [_ w5261]
          tunnel: w5239 -> [_ w5259]
          tunnel: w5238 -> [_ w5257]
          tunnel: w5237 -> [_ w5256]
          tunnel: w5236 -> [_ w5255]
          tunnel: w5235 -> [_ w5254]
          tunnel: w5234 -> [_ w5253]
          tunnel: w5233 -> [_ w5252]
          tunnel: w5232 -> [_ w5251]
          tunnel: w5231 -> [_ w5250]
          frame False {
          }
          frame True {
            n3367 = case shown="True" "Stop saving data + video" {
              frame False {
              }
              frame True {
                n3368 = local write "Save Video"(FALSE ("Save Video")) -> ()
              }
            }
            n3369 = Multiply(x=w5260, y=w5259) -> (x*y=→"Time (s)":dbl)
            n3370 = Less Or Equal?(x=w5260, y=w5268) -> (x <= y?=w5272:bool)
            n3371 = Compound Arithmetic op=OR("Stop Saving", "Abort save 2", "Stop saving data + video") -> (w5264:bool)
            n3372 = Not(x=w5264) -> (.not. x?=w5273:bool)
            n3373 = And(x=w5272, y=w5273) -> (x .and. y?=w5271:bool)
            n3374 = case shown="True" w5271 {
              tunnel: w5274 -> [w5282 w5373]
              tunnel: [0.0 w5376] -> w5267
              tunnel: w5260 -> [_ w5374]
              tunnel: w5268 -> [_ w5375]
              tunnel: w5270 -> [_ w5370]
              tunnel: w5269 -> [_ _]
              tunnel: w5263 -> [w5280 w5363]
              tunnel: w5262 -> [w5279 w5364]
              tunnel: w5261 -> [_ w5362]
              tunnel: w5257 -> [_ w5361]
              tunnel: w5256 -> [_ w5285]
              tunnel: w5255 -> [_ w5354]
              tunnel: w5254 -> [_ w5301]
              tunnel: w5253 -> [w5276 w5318]
              tunnel: w5252 -> [w5277 w5317]
              tunnel: w5251 -> [_ w5314]
              tunnel: w5250 -> [_ w5312]
              frame False {
                w5278 = FALSE
                n3375 = Close File(refnum=w5282) -> ()  [unwired: 1 in, 2 out]
                n3376 = case shown="True" w5279 {
                  tunnel: w5280 -> [_ w5284]
                  frame False {
                  }
                  frame True {
                    n3377 = Close File(refnum=w5284) -> ()  [unwired: 1 in, 2 out]
                  }
                }
                n3378 = case shown="True" w5276 {
                  tunnel: w5277 -> [_ w5283]
                  frame False {
                  }
                  frame True {
                    n3379 = Close File(refnum=w5283) -> ()  [unwired: 1 in, 2 out]
                  }
                }
                n3380 = local write "Raster Scanning..."(w5278) -> ()
                n3381 = local write "Calibrating Trap..."(w5278) -> ()
                n3382 = call <vilib>:"Beep.vi"() -> ()  [unwired: 3 in, 9 out]
                n3383 = local write "Stop Saving"(w5278) -> ()
                "Saving..." <- w5278
              }
              frame True {
                n3384 = local read "Calibrating Trap..."() -> (w5365:bool)
                n3385 = case "Write fl. data" shown="True" w5364 {
                  tunnel: w5363 -> [_ w5399]
                  tunnel: w5362 -> [_ w5398]
                  frame False {
                  }
                  frame True {
                    n3386 = Write to Binary File(file (use dialog)=w5399, data=w5398, 5:FALSE ("prepend array or string size? (T)"), 9:T28."big-endian, network order" ("byte order (0:big-endian, network order)")) -> ()  [unwired: 1 in, 4 out]
                  }
                }
                n3387 = Greater?(x="Save ave N", y=1.0) -> (0:w5368:bool)
                n3388 = Not(x=w5365) -> (.not. x?=w5367:bool)
                n3389 = And(x=w5367, y=w5368) -> (x .and. y?=w5315:bool)
                n3390 = case shown="True" w5315 {
                  tunnel: w5314 -> [w5379 w5390]
                  tunnel: [w5379 w5382] -> w5313
                  tunnel: "Save ave N" -> [_ w5383]
                  frame False {
                  }
                  frame True {
                    w5380 = 2 ("dimension size")
                    n3391 = Array Size(array=w5390) -> (size(s)=w5384:i32)
                    n3392 = Divide(x=w5384, y=w5380) -> (x/y=w5388:dbl)
                    n3393 = Reshape Array(w5390, w5388, w5380) -> (w5389:u64[][])
                    n3394 = Transpose 2D Array(2D array=w5389) -> (transposed array=w5387:u64[][])
                    n3395 = for {
                      tunnel: w5387 -> [w5392] mode=indexing
                      tunnel: [w5391] -> w5381 mode=indexing
                      tunnel: w5383 -> [w5393]
                      workers-P: _ -> [_]
                      n3396 = call "downsample 1D array - U64.vi"("Ave N"=w5393, "Array In"=w5392) -> ("Array Out"=w5391:u64[])  [unwired: 1 in]
                    }
                    n3397 = Transpose 2D Array(2D array=w5381) -> (transposed array=w5386:u64[][])
                    n3398 = Divide(x=w5384, y=w5383) -> (x/y=w5385:dbl)
                    n3399 = Reshape Array(w5386, w5385) -> (w5382:u64[])
                  }
                }
                n3400 = case shown="True" w5315 {
                  tunnel: w5370 -> [w5402 w5414]
                  tunnel: [w5402 w5406] -> w5366
                  tunnel: "Save ave N" -> [_ w5407]
                  tunnel: w5361 -> [_ w5405]
                  frame False {
                  }
                  frame True {
                    n3401 = Array Size(array=w5414) -> (size(s)=w5408:i32)
                    n3402 = Array Size(array=w5405) -> (size(s)=w5404:i32)
                    n3403 = Divide(x=w5408, y=w5404) -> (x/y=w5412:dbl)
                    n3404 = Reshape Array(w5414, w5412, w5404) -> (w5413:i16[][])
                    n3405 = Transpose 2D Array(2D array=w5413) -> (transposed array=w5411:i16[][])
                    n3406 = for {
                      tunnel: w5411 -> [w5417] mode=indexing
                      tunnel: [w5416] -> w5403 mode=indexing
                      tunnel: w5407 -> [w5415]
                      workers-P: _ -> [_]
                      n3407 = call "downsample 1D array - I16.vi"("Ave N"=w5415, "Array In"=w5417) -> ("Array Out"=w5416:i16[])  [unwired: 1 out]
                    }
                    n3408 = Transpose 2D Array(2D array=w5403) -> (transposed array=w5410:i16[][])
                    n3409 = Divide(x=w5408, y=w5407) -> (x/y=w5409:dbl)
                    n3410 = Reshape Array(w5410, w5409) -> (w5406:i16[])
                  }
                }
                n3411 = Index Array(array=w5301, index=2) -> (element=w5302:waveform(dbl))
                n3412 = Index Array(array=w5301, index=1) -> (element=w5335:waveform(dbl))
                n3413 = Index Array(array=w5301, index=0) -> (element=w5337:waveform(dbl))
                n3414 = Unbundle By Name(w5302) -> ("Y"=w5304:dbl[])
                n3415 = Unbundle By Name(w5335) -> ("Y"=w5339:dbl[])
                n3416 = Unbundle By Name(w5337) -> ("Y"=w5347:dbl[])
                n3417 = case "Write trap pos. data" shown="True" w5318 {
                  tunnel: w5317 -> [_ w5395]
                  tunnel: w5313 -> [_ w5394]
                  frame False {
                  }
                  frame True {
                    n3418 = Write to Binary File(file (use dialog)=w5395, data=w5394, 5:FALSE ("prepend array or string size? (T)"), 9:T28."big-endian, network order" ("byte order (0:big-endian, network order)")) -> ()  [unwired: 1 in, 4 out]
                  }
                }
                n3419 = Write to Binary File(file (use dialog)=w5373, data=w5366, 5:FALSE ("prepend array or string size? (T)"), 9:T28."big-endian, network order" ("byte order (0:big-endian, network order)")) -> ()  [unwired: 1 in, 4 out]
                n3420 = feedback #37(w5304) -> (w5305:dbl[])
                n3421 = Build Array (concatenate)(w5305, w5304) -> (w5300:dbl[])
                n3422 = Select(t=w5304, s=w5285, f=w5300) -> (s? t:f=w5290:dbl[])
                n3423 = feedback-in #37(w5290) -> ()
                n3424 = feedback #38(w5339) -> (w5341:dbl[])
                n3425 = Build Array (concatenate)(w5341, w5339) -> (w5340:dbl[])
                n3426 = Select(t=w5339, s=w5285, f=w5340) -> (s? t:f=w5329:dbl[])
                n3427 = feedback-in #38(w5329) -> ()
                n3428 = feedback #39(w5347) -> (w5360:dbl[])
                n3429 = Build Array (concatenate)(w5360, w5347) -> (w5359:dbl[])
                n3430 = Select(t=w5347, s=w5285, f=w5359) -> (s? t:f=w5334:dbl[])
                n3431 = feedback-in #39(w5334) -> ()
                n3432 = Divide(x=w5374, y=w5375) -> (x/y=w5377:dbl)
                n3433 = Multiply(x=w5377, y=100.0) -> (x*y=w5376:dbl)
                n3434 = Build Array(w5334, w5329, w5290) -> (→"Saved APD":dbl[][])
                n3435 = Array Size(array=w5334) -> (size(s)=w5352:i32)
                n3436 = Unbundle By Name(w5354) -> ("Y"=w5358:dbl[])
                n3437 = Subtract(x=w5352, y="N pts to average") -> (x-y=w5287:i32)
                n3438 = Multiply(x="N pts to average", y=u16 2) -> (x*y=w5330:u16)
                n3439 = Subtract(x=w5352, y=w5330) -> (x-y=w5288:i32)
                n3440 = feedback #40(w5358) -> (w5357:dbl[])
                n3441 = Build Array (concatenate)(w5357, w5358) -> (w5356:dbl[])
                n3442 = Select(t=w5358, s=w5285, f=w5356) -> (s? t:f=w5355:dbl[])
                "Trap Delta Graph" <- w5355
                n3443 = feedback-in #40(w5355) -> ()
                n3444 = Array Subset(array=w5334, index=w5287, length="N pts to average") -> (w5351:dbl[])
                n3445 = Array Subset(array=w5334, index=w5288, length="N pts to average") -> (w5350:dbl[])
                n3446 = Array Subset(array=w5329, index=w5287, length="N pts to average") -> (w5332:dbl[])
                n3447 = Array Subset(array=w5329, index=w5288, length="N pts to average") -> (w5331:dbl[])
                n3448 = Array Subset(array=w5290, index=w5287, length="N pts to average") -> (w5299:dbl[])
                n3449 = Array Subset(array=w5290, index=w5288, length="N pts to average") -> (w5298:dbl[])
                n3450 = Index Array(array=w5312, index=0) -> (element=w5310:waveform(dbl))
                n3451 = call-poly <vilib>:"Mean.vi"("X"=w5351) -> ("mean"=w5349:dbl)  [unwired: 1 out]
                n3452 = call-poly <vilib>:"Mean.vi"("X"=w5332) -> ("mean"=w5328:dbl)  [unwired: 1 out]
                n3453 = call-poly <vilib>:"Mean.vi"("X"=w5350) -> ("mean"=w5348:dbl)  [unwired: 1 out]
                n3454 = call-poly <vilib>:"Mean.vi"("X"=w5331) -> ("mean"=w5327:dbl)  [unwired: 1 out]
                n3455 = call-poly <vilib>:"Mean.vi"("X"=w5299) -> ("mean"=w5297:dbl)  [unwired: 1 out]
                n3456 = call-poly <vilib>:"Mean.vi"("X"=w5298) -> ("mean"=w5296:dbl)  [unwired: 1 out]
                n3457 = Unbundle By Name(w5310) -> ("Y"=w5308:dbl[])
                n3458 = Subtract(x=w5328, y=w5327) -> (x-y=w5319:dbl)
                "Delta Fl. 2" <- w5319
                n3459 = Subtract(x=w5297, y=w5296) -> (x-y=w5291:dbl)
                "Delta Fl. 3" <- w5291
                n3460 = Subtract(x=w5349, y=w5348) -> (x-y=w5346:dbl)
                "Delta Fl. 1" <- w5346
                n3461 = feedback #41(w5308) -> (w5307:dbl[])
                n3462 = Build Array (concatenate)(w5307, w5308) -> (w5309:dbl[])
                n3463 = Initialize Array(w5346, 1 ("dimension size")) -> (w5343:dbl[])
                n3464 = Initialize Array(w5319, 1 ("dimension size")) -> (w5324:dbl[])
                n3465 = Initialize Array(w5291, 1 ("dimension size")) -> (w5293:dbl[])
                n3466 = Select(t=w5308, s=w5285, f=w5309) -> (s? t:f=w5306:dbl[])
                "Saved trap pos" <- w5306
                n3467 = feedback-in #41(w5306) -> ()
                n3468 = feedback #42(w5343) -> (w5344:dbl[])
                n3469 = Build Array (concatenate)(w5344, w5343) -> (w5342:dbl[])
                n3470 = feedback #43(w5324) -> (w5325:dbl[])
                n3471 = feedback #44(w5293) -> (w5294:dbl[])
                n3472 = Build Array (concatenate)(w5325, w5324) -> (w5323:dbl[])
                n3473 = Build Array (concatenate)(w5294, w5293) -> (w5292:dbl[])
                n3474 = Select(t=w5343, s=w5285, f=w5342) -> (s? t:f=w5322:dbl[])
                n3475 = feedback-in #42(w5322) -> ()
                n3476 = Select(t=w5324, s=w5285, f=w5323) -> (s? t:f=w5321:dbl[])
                n3477 = feedback-in #43(w5321) -> ()
                n3478 = Select(t=w5293, s=w5285, f=w5292) -> (s? t:f=w5286:dbl[])
                n3479 = feedback-in #44(w5286) -> ()
                n3480 = Build Array(w5322, w5321, w5286) -> (→"Save APD Deriv":dbl[][])
              }
            }
            "Progress" <- w5267
            "Progress 2" <- w5267
          }
        }
      }
    }
    n3481 = local read "wait to reset values"() -> (w3891:bool)
    n3482 = Not(x=w3889) -> (.not. x?=w3892:bool)
    n3483 = And(x=w3892, y=w3891) -> (x .and. y?=w3893:bool)
    n3484 = case "Part of MCL raster scanning: returns to initial positions after scan done" shown="True" w3893 {
      tunnel: w3632 -> [w4790 w4797]
      tunnel: [w4790 w4796] -> w3895
      tunnel: w3631 -> [w4789 w4795]
      tunnel: [w4789 w4794] -> w3890
      frame False {
      }
      frame True {
        w4805 = 10.0 ("y")
        w4804 = 32767.0 ("y")
        # "to return scan values\nafter a synchronous \nAOM scan"
        n3485 = local read "AO2"() -> (w4798:dbl)
        n3486 = local read "AO1"() -> (w4799:dbl)
        n3487 = local write "wait to reset values"(FALSE ("wait to reset values")) -> ()
        n3488 = Multiply(x=w4799, y=w4804) -> (x*y=w4801:dbl)
        n3489 = Multiply(x=w4798, y=w4804) -> (x*y=w4803:dbl)
        n3490 = Divide(x=w4801, y=w4805) -> (x/y=w4800:dbl)
        n3491 = Divide(x=w4803, y=w4805) -> (x/y=w4802:dbl)
        n3492 = To Word Integer(number=w4800) -> (16bit integer=w4806:i16)
        n3493 = To Word Integer(number=w4802) -> (16bit integer=w4807:i16)
        n3494 = local read "Total Counts (ticks)"() -> (w4791:u16)
        n3495 = xnode "Read/Write Control"("FPGA VI Reference In"=w4797, "error in"=w4795, "AO1"=w4806, "AO2"=w4807, "MCL count"=w4791) -> ("FPGA VI Reference Out"=w4796:T20, "error out"=w4794:errorcluster)
        n3496 = local read "Scan Range (V)\n(of steps)"() -> (w4792:dbl)
        n3497 = property on="Scan Range (V)\n(of steps)" class="DigNum (strict)"("Val(Sgnl)"=w4792) -> ()  [unwired: 2 in, 2 out]
      }
    }
    n3498 = node-c288() -> ()  [unwired: 2 out]
  }
  n3499 = node-c288(w21) -> ()  [unwired: 1 out]
  n3500 = node-c288(w65) -> ()  [unwired: 1 out]
  n3501 = node-c288(w67) -> ()  [unwired: 1 out]
  n3502 = node-c288(w53) -> ()  [unwired: 1 out]
  n3503 = property on="Saved trap pos" class="WFGraph (strict)"("Visible"=FALSE) -> ()  [unwired: 2 in, 2 out]
  n3504 = property on="Trap Delta Graph" class="WFGraph (strict)"("Visible"=TRUE) -> ()  [unwired: 2 in, 2 out]
  n3505 = local write "Trap pos"(FALSE ("Trap pos")) -> ()
  n3506 = disable-structure shown="Disabled" {
    disable-tunnel: w57 -> [w5419 _]
    disable-tunnel: w56 -> [w5418 _]
    frame Disabled {
      n3507 = VISA Close(VISA resource name=w5419, error in (no error)=w5418) -> (error out=w5420:errorcluster)
      n3508 = call <vilib>:"Simple Error Handler.vi"("error in (no error)"=w5420) -> ()  [unwired: 1 in, 8 out]
    }
    frame Enabled {
    }
  }
  n3509 = node-c288(w63) -> ()  [unwired: 1 out]
  n3510 = node-c288(w72) -> ()  [unwired: 1 out]
  n3511 = flat-sequence {
    tunnel: w79 -> [w5424]
    tunnel: w80 -> [w5425]
    tunnel: [w5423] -> w78
    tunnel: [w5422] -> w77
    tunnel: w76 -> [_]
    tunnel: w74 -> [_]
    tunnel: w69 -> [_]
    tunnel: w78 -> [w5426]
    tunnel: w77 -> [w5427]
    frame #0 {
      w5421 = FALSE ("AI to FIFO")
      n3512 = xnode "Read/Write Control"("FPGA VI Reference In"=w5425, "error in"=w5424, "AI to FIFO"=w5421, "APD to FIFO"=w5421) -> ("FPGA VI Reference Out"=w5423:T20, "error out"=w5422:errorcluster)
    }
    frame #1 {
      n3513 = xnode "Close FPGA VI Reference"("FPGA VI Reference In"=w5426, "error in"=w5427) -> ("error out"=→"error out":errorcluster)
    }
  }
